vi "Sync clocks.vi"   [LabVIEW 2023]
uses:
  <vilib>/Utility/error.llb/DialogType.ctl
  <vilib>/DAQmx/write.llb/DAQmx Write (Analog 2D DBL NChan NSamp).vi
  <vilib>/DAQmx/read.llb/DAQmx Read (Analog 2D DBL NChan NSamp).vi
  <vilib>/DAQmx/create/channels.llb/DAQmx Create Channel (AI-Voltage-Basic).vi
  <vilib>/DAQmx/configure/timing.llb/DAQmx Timing (Sample Clock).vi
  <vilib>/DAQmx/configure/trigger.llb/DAQmx Reference Trigger (Digital Edge).vi
  <vilib>/DAQmx/create/channels.llb/DAQmx Create Channel (AO-Voltage-Basic).vi
  <vilib>/DAQmx/configure/trigger.llb/DAQmx Start Trigger (Digital Edge).vi
  <vilib>/DAQmx/configure/trigger.llb/DAQmx Start Trigger (Time).vi
  <vilib>/DAQmx/configure/trigger.llb/DAQmx Start Trigger (Analog Edge).vi
  <vilib>/DAQmx/miscellaneous.llb/DAQmx Fill In Error Info.vi
  <resource>/objmgr/daqmx.rc
types:
  T1 = enum16{"open", "replace", "create", "open or create", "replace or create", "replace or create with confirmation"}
  T2 = enum16{"big-endian, network order", "native, host order", "little-endian"}
  T3 = typedef "DialogType.ctl" = u16
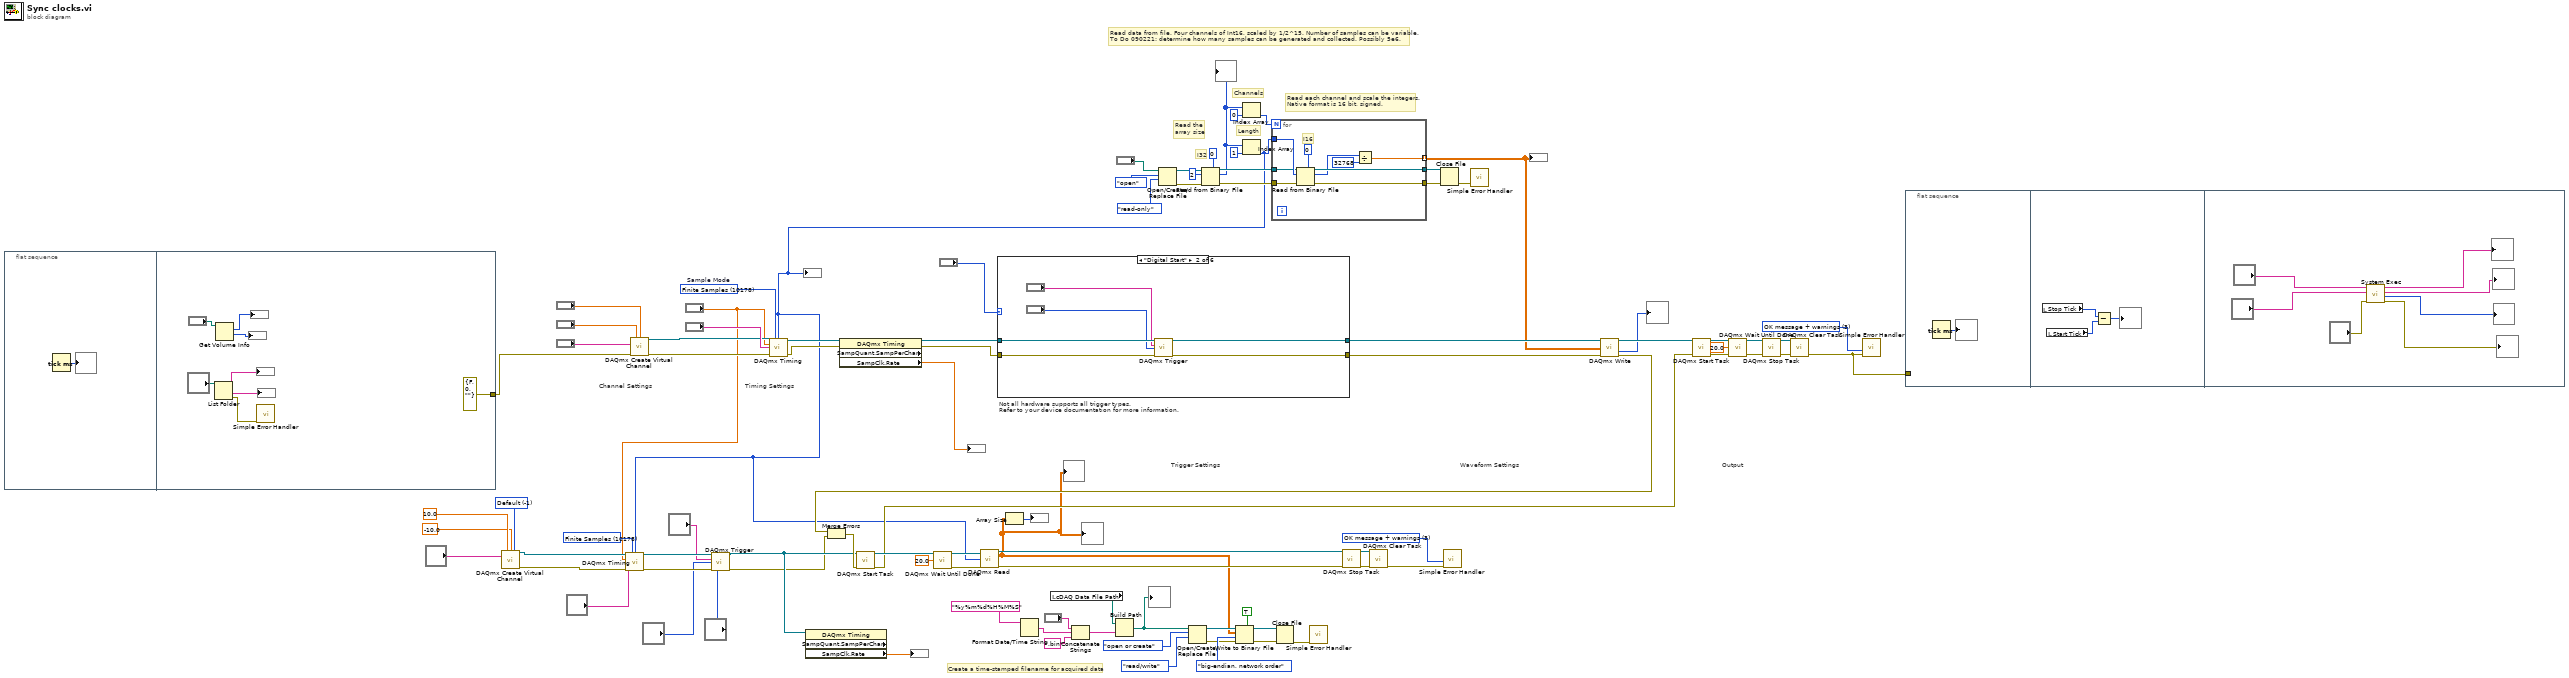
[diagram p0: block diagram]
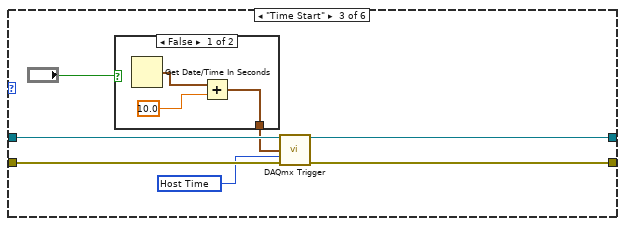
[diagram p3: hidden frame]
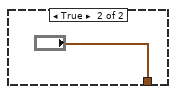
[diagram p4: hidden frame]
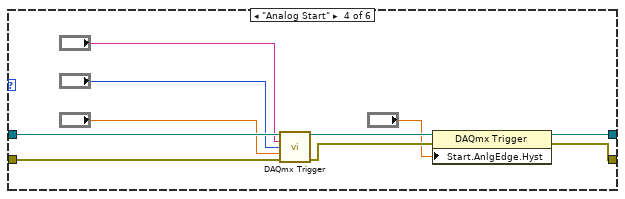
[diagram p5: hidden frame]
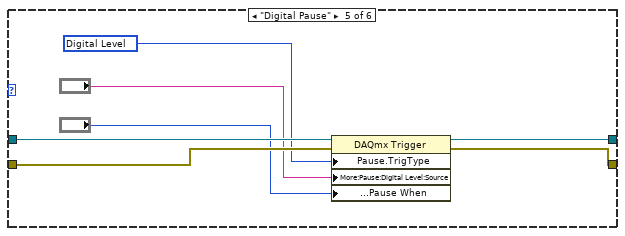
[diagram p6: hidden frame]
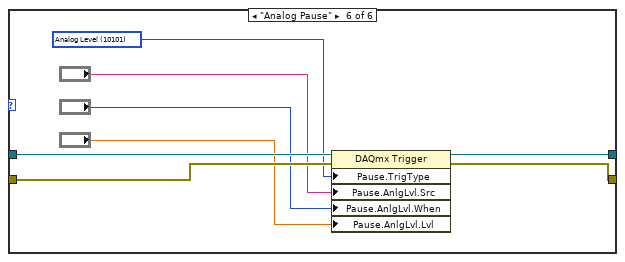
[diagram p7: hidden frame]
diagram:
  w57 = 10178 items=["Finite Samples"=10178, "Continuous Samples"=10123, "Hardware Timed Single Point"=12522] ("sample mode")
  w64 = T3 3 items=["no dialog", "OK message", "continue or stop message", "OK message + warnings", "continue/stop + warnings"] ("type of dialog (OK msg:1)")
  w69 = -1 items=["Default"=-1, "RSE"=10083, "NRSE"=10078, "Differential"=10106, "Pseudodifferential"=12529] ("input terminal configuration")
  w78 = T3 3 items=["no dialog", "OK message", "continue or stop message", "OK message + warnings", "continue/stop + warnings"] ("type of dialog (OK msg:1)")
  w91 = 10178 items=["Finite Samples"=10178, "Continuous Samples"=10123, "Hardware Timed Single Point"=12522]  # Sample Mode
  # "Create a time-stamped filename for acquired data"
  # "Read each channel and scale the integers.\nNative format is 16 bit, signed."
  # "Length"
  # "Channels"
  # "Read the \narray size"
  # "Read data from file. Four channels of Int16, scaled by 1/2^15. Number of samples can be variable. \nTo Do 090221: determine how many samples can be generated and collected. Possibly 5e6."
  # "I32"
  # "Trigger Settings"
  # "Not all hardware supports all trigger types.\nRefer to your device documentation for more information."
  # "Output"
  # "Waveform Settings"
  # "Timing Settings"
  # "Channel Settings"
  n1 = flat-sequence {
    tunnel: [errorcluster {"status"=FALSE, "code"=0, "source"=""} ("error constant")] -> w41
    frame #0 {
      n2 = Tick Count (ms)() -> (millisecond timer value=→"?":u32)
    }
    frame #1 {
      n3 = List Folder(path="?") -> (filenames=→"?":string[], folder names=→"?":string[], error out=w97:errorcluster)  [unwired: 3 in, 1 out]
      n4 = Get Volume Info(11:"?") -> (1:→"?":i64, 2:→"?":i64)  [unwired: 1 in, 4 out]
      n5 = call <vilib>:"Simple Error Handler.vi"("error in (no error)"=w97) -> ()  [unwired: 4 in, 5 out]
    }
  }
  n6 = call-poly <vilib>:"DAQmx Create Virtual Channel.vi"("maximum value"=10.0, "minimum value"=-10.0, "input terminal configuration"=w69, "physical channels"="?") -> ("task out"=w63:refnum<k21>, "error out"=w60:errorcluster)  [unwired: 10 in]
  n7 = call-poly <vilib>:"DAQmx Create Virtual Channel.vi"("maximum value"="?", "minimum value"="?", "physical channels"="?", "error in"=w41) -> ("task out"=w73:refnum<k21>, "error out"=w90:errorcluster)  [unwired: 10 in]
  n8 = Format Date/Time String(time format string (%c)="%y%m%d%H%M%S") -> (date/time string=w37:string)  [unwired: 2 in]
  n9 = local read "cDAQ Data File Path"() -> (w40:path)
  n10 = Concatenate Strings("?", w37, ".bin" ("string")) -> (w35:string)
  n11 = Build Path(base path=w40, name or relative path=w35) -> (appended path=w34:path)
  "?" <- w34
  n12 = Open/Create/Replace File(file path (use dialog)="?", operation (0:open)=T1."open", access (0:read/write)=enum16{"read/write", "read-only", "write-only"}."read-only") -> (refnum out=w22:refnum<file>, error out=w21:errorcluster)  [unwired: 3 in, 1 out]
  n13 = Open/Create/Replace File(file path (use dialog)=w34, operation (0:open)=T1."open or create", access (0:read/write)=enum16{"read/write", "read-only", "write-only"}."read/write") -> (refnum out=w31:refnum<file>, error out=w29:errorcluster)  [unwired: 3 in, 1 out]
  n14 = Read from Binary File(5:0, 8:w21, 10:2 ("count (1)"), 11:w22) -> (0:w15:errorcluster, 2:w8:i32[], 3:w13:refnum<file>)  [unwired: 2 in, 1 out]
  "?" <- w8
  n15 = Index Array(array=w8, index=0) -> (element=w17:i32)
  n16 = Index Array(array=w8, index=1) -> (element=w3:i32)
  "?" <- w3
  n17 = call-poly <vilib>:"DAQmx Timing.vi"("task/channels in"=w63, "sample mode"=w57, "samples per channel"=w3, "rate"="?", "source"="?", "error in"=w60) -> ("task out"=w50:refnum<k21>, "error out"=w48:errorcluster)  [unwired: 8 in]
  n18 = call-poly <vilib>:"DAQmx Trigger.vi"("task/channels in"=w50, "source"="?", "edge"="?", "error in"=w48, "pretrigger samples per channel"="?") -> ("task out"=w49:refnum<k21>, "error out"=w47:errorcluster)  [unwired: 9 in]
  n19 = call-poly <vilib>:"DAQmx Timing.vi"("task/channels in"=w73, "sample mode"=w91, "samples per channel"=w3, "rate"="?", "source"="?", "error in"=w90) -> ("task out"=w93:refnum<k21>, "error out"=w92:errorcluster)  [unwired: 8 in]
  n20 = property class="DAQmx Timing" props=["SampQuant.SampPerChan", "SampClk.Rate"](reference=w49) -> ("SampClk.Rate"=→"?":dbl)  [unwired: 1 in, 3 out]
  n21 = property class="DAQmx Timing" props=["SampQuant.SampPerChan", "SampClk.Rate"](reference=w93, error in=w92) -> (reference out=w74:refnum<k21>, error out=w75:errorcluster, "SampClk.Rate"=→"?":dbl)  [unwired: 1 out]
  n22 = case shown="\"Digital Start\"" "?" {
    tunnel: w74 -> [w104 w110 w117 w131 w138 w146]
    tunnel: w75 -> [w103 w109 w116 w130 w135 w143]
    tunnel: [w104 w108 w115 w128 w137 w145] -> w76
    tunnel: [w103 w107 w114 w127 w136 w144] -> w24
    frame "No Trigger", Default {
    }
    frame "Digital Start" {
      n23 = call-poly <vilib>:"DAQmx Trigger.vi"("task/channels in"=w110, "source"="?", "edge"="?", "error in"=w109) -> ("task out"=w108:refnum<k21>, "error out"=w107:errorcluster)  [unwired: 10 in]
    }
    frame "Time Start" {
      w113 = 16126 items=["Host Time"=16126, "I/O Device Time"=16127] ("timescale")
      n24 = case shown="False" "?" {
        tunnel: [w119 "?"] -> w111
        frame False {
          n25 = Get Date/Time In Seconds() -> (seconds since 1Jan1904=w120:timestamp)
          n26 = Add(x=w120, y=10.0) -> (x+y=w119:timestamp)
        }
        frame True {
        }
      }
      n27 = call-poly <vilib>:"DAQmx Trigger.vi"("task/channels in"=w117, "when"=w111, "timescale"=w113, "error in"=w116) -> ("task out"=w115:refnum<k21>, "error out"=w114:errorcluster)  [unwired: 10 in]
    }
    frame "Analog Start" {
      n28 = call-poly <vilib>:"DAQmx Trigger.vi"("task/channels in"=w131, "source"="?", "slope"="?", "level"="?", "error in"=w130) -> ("task out"=w126:refnum<k21>, "error out"=w125:errorcluster)  [unwired: 9 in]
      n29 = property class="DAQmx Trigger"(reference=w126, error in=w125, "Start.AnlgEdge.Hyst"="?") -> (reference out=w128:refnum<k21>, error out=w127:errorcluster)
    }
    frame "Digital Pause" {
      w134 = 10152 items=["Analog Level"=10101, "Analog Window"=10103, "Digital Level"=10152, "Digital Pattern"=10398, "None"=10230] ("Pause.TrigType")
      n30 = property class="DAQmx Trigger"(reference=w138, error in=w135, "Pause.TrigType"=w134, "More:Pause:Digital Level:Source"="?", "More:Pause:Digital Level:Pause When"="?") -> (reference out=w137:refnum<k21>, error out=w136:errorcluster)
    }
    frame "Analog Pause" {
      w142 = 10101 items=["Analog Level"=10101, "Analog Window"=10103, "Digital Level"=10152, "Digital Pattern"=10398, "None"=10230] ("Pause.TrigType")
      n31 = property class="DAQmx Trigger"(reference=w146, error in=w143, "Pause.TrigType"=w142, "Pause.AnlgLvl.Src"="?", "Pause.AnlgLvl.When"="?", "Pause.AnlgLvl.Lvl"="?") -> (reference out=w145:refnum<k21>, error out=w144:errorcluster)
    }
  }
  n32 = for {
    N: w17 -> [_]
    tunnel: w3 -> [w155]
    tunnel: w15 -> [w153]
    tunnel: [w152] -> w14
    tunnel: w13 -> [w151]
    tunnel: [w150] -> w12
    tunnel: [w147] -> w9 mode=indexing
    # "I16"
    n33 = Read from Binary File(5:i16 0, 8:w153, 10:w155, 11:w151) -> (0:w152:errorcluster, 2:w149:i16[], 3:w150:refnum<file>)  [unwired: 2 in, 1 out]
    n34 = Divide(x=w149, y=32768) -> (x/y=w147:dbl[])
  }
  "?" <- w9
  n35 = Close File(refnum=w12, error in=w14) -> (error out=w2:errorcluster)  [unwired: 1 out]
  n36 = call <vilib>:"Simple Error Handler.vi"("error in (no error)"=w2) -> ()  [unwired: 4 in, 5 out]
  n37 = call-poly <vilib>:"DAQmx Write.vi"("task/channels in"=w76, "data"=w9, "error in"=w24) -> ("task out"=w85:refnum<k21>, "number of samples written per channel"=→"?":u32, "error out"=w56:errorcluster)  [unwired: 10 in]
  n38 = Merge Errors(w56, w47) -> (w55:errorcluster)
  n39 = call <vilib>:"DAQmx Start Task.vi"("task/channels in"=w49, "error in"=w55) -> ("task out"=w67:refnum<k21>, "error out"=w54:errorcluster)  [unwired: 12 in]
  n40 = call <vilib>:"DAQmx Wait Until Done.vi"("task/channels in"=w67, "timeout (sec)"=20.0) -> ("task out"=w62:refnum<k21>, "error out"=w59:errorcluster)  [unwired: 12 in]
  n41 = call-poly <vilib>:"DAQmx Read.vi"("task/channels in"=w62, "number of samples per channel"=w3, "error in"=w59) -> ("task out"=w61:refnum<k21>, "data"=w4:dbl[][], "error out"=w58:errorcluster)  [unwired: 10 in]
  "?" <- w4
  "?" <- w4
  n42 = Array Size(array=w4) -> (size(s)=→"?":i32[])
  n43 = Write to Binary File(file (use dialog)=w31, data=w4, error in=w29, 5:TRUE ("prepend array or string size? (T)"), 9:T2."big-endian, network order" ("byte order (0:big-endian, network order)")) -> (refnum out=w26:refnum<file>, error out=w27:errorcluster)  [unwired: 1 in, 1 out]
  n44 = Close File(refnum=w26, error in=w27) -> (error out=w25:errorcluster)  [unwired: 1 out]
  n45 = call <vilib>:"Simple Error Handler.vi"("error in (no error)"=w25) -> ()  [unwired: 4 in, 5 out]
  n46 = call <vilib>:"DAQmx Stop Task.vi"("task/channels in"=w61, "error in"=w58) -> ("task out"=w66:refnum<k21>, "error out"=w65:errorcluster)  [unwired: 12 in]
  n47 = call <vilib>:"DAQmx Clear Task.vi"("task in"=w66, "error in"=w65) -> ("error out"=w68:errorcluster)  [unwired: 13 in]
  n48 = call <vilib>:"Simple Error Handler.vi"("type of dialog (OK msg:1)"=w64, "error in (no error)"=w68) -> ()  [unwired: 3 in, 5 out]
  n49 = call <vilib>:"DAQmx Start Task.vi"("task/channels in"=w85, "error in"=w54) -> ("task out"=w84:refnum<k21>, "error out"=w83:errorcluster)  [unwired: 12 in]
  n50 = call <vilib>:"DAQmx Wait Until Done.vi"("task/channels in"=w84, "timeout (sec)"=20.0, "error in"=w83) -> ("task out"=w80:refnum<k21>, "error out"=w79:errorcluster)  [unwired: 11 in]
  n51 = call <vilib>:"DAQmx Stop Task.vi"("task/channels in"=w80, "error in"=w79) -> ("task out"=w82:refnum<k21>, "error out"=w81:errorcluster)  [unwired: 12 in]
  n52 = call <vilib>:"DAQmx Clear Task.vi"("task in"=w82, "error in"=w81) -> ("error out"=w1:errorcluster)  [unwired: 13 in]
  n53 = call <vilib>:"Simple Error Handler.vi"("type of dialog (OK msg:1)"=w78, "error in (no error)"=w1) -> ()  [unwired: 3 in, 5 out]
  n54 = flat-sequence {
    tunnel: w1 -> [_]
    frame #0 {
      n55 = Tick Count (ms)() -> (millisecond timer value=→"?":u32)
    }
    frame #1 {
      n56 = local read "Stop Tick"() -> (w159:u32)
      n57 = local read "Start Tick"() -> (w158:u32)
      n58 = Subtract(x=w159, y=w158) -> (x-y=→"?":u32)
    }
    frame #2 {
      n59 = call <vilib>:"System Exec.vi"("error in (no error)"="?", "standard input"="?", "command line"="?") -> ("error out"=→"?":errorcluster, "return code"=→"?":i32, "standard error"=→"?":string, "standard output"=→"?":string)  [unwired: 5 in]
    }
  }
